vi "generate and convert rnd 1,2,3-D arrays.vi"(0 "dims":i32, 1 "numeric type const":T1, 5 "Tag":string, 9 "sizes":T4, 11 "error in (no error)":errorcluster) -> (2 "current timepoint":dbl, 3 "Array 1D":cdb[](array[numeric]), 4 "Array 2D":cdb[][](array[numeric]), 6 "Array 3D":cdb[][][](array[numeric]), 8 "bytes":i32, 10 "array as variant":variant, 12 "element size (bytes)":u8, 13 "delta t (s)":dbl, 14 "Bindata & descr out":T2, 15 "error out":errorcluster)   [LabVIEW 2018, in "LV2Julia_examples.lvlib"] (continued)
  1ec9265c-e1ac-4cb5-8500-03f8ca54a804.vi/ab8334bc-80fe-49a7-aeaa-72d4d4d986e9.vi/b9ff3e0a-05c7-4d11-a75b-368fec092445.vi/274aa64d-7dbc-4001-99d2-75c7e6616095.vi
  1ec9265c-e1ac-4cb5-8500-03f8ca54a804.vi/96353e94-dd23-4035-8dd4-90333fc8a4d3.vi/f4ce16f9-675e-447e-8c5f-32c7ef14206e.vi/2ab18f9f-d25e-4d6f-a422-5d1976ace012.vi
  1ec9265c-e1ac-4cb5-8500-03f8ca54a804.vi/167585a2-6b26-4dd4-a205-ebd7312b44a1.vi/4f7bf506-ab24-41ce-b71a-8160a5476407.vi/342633a8-57f8-4cc5-bcb8-03c25e82ca19.vi
  9cd03b83-d5bc-4a7f-9dd3-ef622f64ee30.vi/c26303ed-4f99-4591-9769-7eebad8d47fd.vi/1b763a9f-5ce5-41ba-bc7f-9f995f4d2b4d.vi/1789e023-f5c5-4665-87e0-2a6614aebc85.vi
  9cd03b83-d5bc-4a7f-9dd3-ef622f64ee30.vi/401e3ff0-0d76-40e6-a2f4-d101c51ec70e.vi/66e2e3b0-dc28-4f05-a834-250e6508c857.vi/552213f3-3728-4a7f-86dc-322237ece7cd.vi
  9cd03b83-d5bc-4a7f-9dd3-ef622f64ee30.vi/b4056afe-3c0d-4dbc-a3cd-b11ce2b05076.vi/40f3e5bb-f60e-451c-8b00-4309ab568451.vi/4e93cb2a-2fda-4bca-9a11-733b7b362d86.vi
  ee83ef70-773d-469c-ba23-25239dc81b12.vi/c87a68b0-2172-4a67-a6f0-f210c7451bd3.vi/84a80026-1c80-486c-8d92-8831a7df5ff3.vi/628bd820-375e-420b-b97f-d572ea6ad967.vi
  ee83ef70-773d-469c-ba23-25239dc81b12.vi/4135ce50-1702-49d5-b7b5-9d498c87c660.vi/d1bc0e7f-a379-4ff9-bf17-9e41a0f46a57.vi/980bb05f-dadf-4b86-b249-59f560e02473.vi
  ee83ef70-773d-469c-ba23-25239dc81b12.vi/9914fa42-08c7-43b8-a27e-b62889b56e78.vi/5de439e2-5012-4648-894c-bb1b9ad5bb26.vi/d9b0be4b-4247-47fe-91b4-82206086a95d.vi
  fca8e823-b190-45b9-9fbf-0f97a3b8de28.vi/a46cdcc9-52d0-4030-83dd-4ce08d19186e.vi/90bccda5-6ac7-4d46-9afb-e6399bdb2e1f.vi/078c7d38-6c67-4563-ab55-40eabe55752b.vi
  fca8e823-b190-45b9-9fbf-0f97a3b8de28.vi/4dbc5799-ec76-42b3-bb12-e906c396b96b.vi/ec007a79-76e9-41e5-8892-0302a9e6b40b.vi/301a90ca-8247-4ad5-ba2b-678751a04883.vi
  fca8e823-b190-45b9-9fbf-0f97a3b8de28.vi/cb420030-84f1-4efb-80b2-f5620303c743.vi/2c209796-9244-4d59-a9f5-eb5b4e6512ff.vi/25dea5f7-681f-4e0e-85cf-2491529aaee2.vi
  e5719774-7c0b-4606-b38f-adf2a3fe0ebf.vi/e04a025a-b044-48ec-9ce3-537d6650ec9f.vi/be8c913f-5955-4425-929d-934409af2b49.vi/d34738e1-42d1-4bf7-9a84-ddff0b876cf5.vi
  e5719774-7c0b-4606-b38f-adf2a3fe0ebf.vi/6399dd36-c1e6-41ee-ae47-d998c15f331f.vi/49d2f734-92bf-43e0-a325-d114aa2d52b5.vi/f6894c85-aa94-43f5-b724-8f72549e5cda.vi
  e5719774-7c0b-4606-b38f-adf2a3fe0ebf.vi/c5e050e8-c7cb-4905-8055-5f2d77b4ebae.vi/22426407-5a39-4ae1-b419-51b886c4e6cc.vi/0f5aa2a8-f382-4938-b1c0-af64f89efd9d.vi
  0f763169-7436-48fd-a14e-d5e7c7a3701c.vi/4318b9fa-7e96-4320-ad14-e58bf08cbdca.vi/ec80edef-ad4d-481c-bae0-ad236ad91d17.vi/99c98c4d-5a9d-4194-a764-b16bcb65aadc.vi
  0f763169-7436-48fd-a14e-d5e7c7a3701c.vi/42337aaa-b56a-45f8-8fc1-26a400602ff7.vi/853c4e43-66a7-4fd6-8a67-725115d20b02.vi/e1340f66-9321-4958-baeb-f40ca0670b2a.vi
  0f763169-7436-48fd-a14e-d5e7c7a3701c.vi/6ec92a7e-3200-4835-a3af-72f6deb2a7de.vi/d7fa0239-54ab-48c8-b35d-0719727c3c46.vi/a08a90ec-3f4e-4bf9-bfc8-c8b0dc2424f1.vi
  85ae8d2b-1833-426f-a7e3-0aa59edb462e.vi/8e85eddd-eeb1-48c7-aa0c-acb2476f15c2.vi/08ea7271-58f7-4381-bb13-89612bf68987.vi/c319c975-6598-4c49-9112-e1ac8bec7b87.vi/58ceea13-0e9b-4af9-9c64-6ddff0cfcc70.vi
  85ae8d2b-1833-426f-a7e3-0aa59edb462e.vi/af9a9771-594c-4ddf-b656-7825023e47e7.vi/a558cd4b-dbd0-4514-827e-24ca6e6b3a91.vi/23666670-5fa0-4551-929a-5078f8c88eb4.vi/ef739d47-3b07-40f6-99d3-e1375b6b8ec0.vi
  85ae8d2b-1833-426f-a7e3-0aa59edb462e.vi/f9469cc9-c20f-42ad-af32-5d4df993a375.vi/8c409728-000f-45f8-9ccd-ee15c7ed8521.vi/af52c658-7aca-4654-a19b-bdc00d5bce4f.vi/47bd8f68-fb6a-411a-b5e7-9fbf321a4e11.vi
  b7a12c6c-f00d-43e6-9642-9243e32b2058.vi/0ada88ee-c4f2-4d17-bb7a-74a21d7765a4.vi/69bbc40a-c36a-4917-aaee-edada7b7b8d7.vi/c11b2df1-177a-40a7-9ba6-98232f8d7f99.vi/7a8a583f-169c-44ac-bc13-e659061e41ae.vi
  b7a12c6c-f00d-43e6-9642-9243e32b2058.vi/502a5a5e-5782-46f9-888a-3583fb3fbf86.vi/571e470d-9707-4b89-9631-5b8d9304f753.vi/e1749920-efd2-42e0-885b-7fb6c4c5ab43.vi/a2170132-eaf3-4ab4-8383-804d572dbb60.vi
  b7a12c6c-f00d-43e6-9642-9243e32b2058.vi/963765af-ec1a-4af6-8576-dda3e1cb1b45.vi/a9e7bee4-94d8-4d8e-b190-a2971037c66e.vi/1f67fc8e-8653-4e8b-a6c2-2cf9980ddd08.vi/c5ad99fd-dcdc-41c3-9a54-18b338f6f827.vi
  ba780daf-ef06-44ce-bff3-6c34795b2ca8.vi/faf0b0c0-115a-4e37-90b8-e50dcc4168bc.vi/ff37c594-a005-47f5-bb34-4c70a0126acb.vi/c6e85278-50f0-4f6a-9193-dc1bcd0ef70f.vi/a77b55b7-d308-4fb3-aa63-6804bc56a6d7.vi
  ba780daf-ef06-44ce-bff3-6c34795b2ca8.vi/3ee41887-da2e-4051-ad5a-82b4c75e16db.vi/43312af0-9a58-49ee-9340-b8aa225bd272.vi/3269ca27-2cba-45df-9346-92c5d96bd6fc.vi/8956672e-b90e-41c9-981a-392c13e15a59.vi
  ba780daf-ef06-44ce-bff3-6c34795b2ca8.vi/440f1969-f94a-49e7-92dd-969720926e87.vi/1b453ea8-962a-4255-a994-0cbca27764d4.vi/f62144a5-f5db-4e00-a07d-a8ab4245d2e0.vi/63c49d2f-fa43-4a67-9b23-eadd08c82c33.vi
  0827bc69-4216-4d70-a1a4-4bfc71e08fdd.vi/261e91eb-d6ba-4368-8adb-b056b6d5af16.vi/d1f6d98c-0505-4e61-9b8c-a3eed1ff26ed.vi/7d30ac35-157d-4fcc-9b6f-176c22041dd3.vi/6365f774-6091-4c03-be79-b53c3a463edd.vi
  0827bc69-4216-4d70-a1a4-4bfc71e08fdd.vi/1cb40332-89ee-4e85-bdd1-f055d6e9593b.vi/3667db32-83c2-4485-8485-501a99b88cfe.vi/a5ed325d-485e-44f9-b4a5-b94842094a7d.vi/bbb4fa19-a19e-4b4f-a972-0fad6acc7987.vi
  0827bc69-4216-4d70-a1a4-4bfc71e08fdd.vi/2aac3158-face-4bd6-b9ad-b375428daa75.vi/10b5fca0-4c2a-4c9a-8b53-fb3dcff5ab00.vi/83375121-0e11-44d4-aa51-0de5076e5d92.vi/8d656ec8-2c6e-4c54-b472-f9621b7bc254.vi
  31a52eb7-4f60-473e-a06e-05ec52e66b84.vi/833f7a80-f94e-40d2-8863-3d22036f4c05.vi/de0d82be-3b4d-4b69-b774-1ee66ef3b500.vi/3a45cae5-de8a-427f-805d-7805f64916c3.vi/779167f3-7191-404e-9479-d306974a1702.vi
  31a52eb7-4f60-473e-a06e-05ec52e66b84.vi/4dc64207-d105-4bdf-b337-3f5f3ae1db54.vi/7b76e6e9-99fc-48fe-88e5-663e33f1532b.vi/06f57519-d6ad-4a96-9600-46d432553020.vi/86d7e16d-a525-46dc-8e9b-8a765bb4fd8a.vi
  31a52eb7-4f60-473e-a06e-05ec52e66b84.vi/caebaab9-5afa-4ebd-88ee-492fb4ee9da6.vi/ae77f17b-7a63-49d8-8677-2eb378eecda7.vi/07361902-21c8-49bd-b0fa-bce76e827913.vi/6519da9f-9d74-43b4-95c4-6905f871aa2b.vi
  be087227-1c24-4c50-b280-a6b288463f93.vi/77d648b1-c2bd-47e8-9d98-d5979e8947bd.vi/eb2ac645-ddc7-47bc-9d8b-75952129f04e.vi/90e6bd1a-94b1-4e35-a711-208e6fb95ce0.vi/4cf44929-3de7-4a16-8e6d-ba3e81e4c27d.vi
  be087227-1c24-4c50-b280-a6b288463f93.vi/9db986cd-cad9-4629-9f04-d611e563b09c.vi/b1da1a18-7165-4dcd-a4ff-b5fd07c18a7e.vi/e9ab5a05-9916-45bc-bc4c-428d98bb0cc0.vi/87e8c9e4-61f1-41fd-91f0-278c7c3c04e0.vi
  be087227-1c24-4c50-b280-a6b288463f93.vi/67544f08-8803-4e76-831f-e149eee3dcfb.vi/541c202c-62e7-4b26-a949-153a4b69c346.vi/04e1edd0-f714-4231-8a6f-30cd0f5f9b80.vi/a19ed12b-7c03-4017-abb4-26d2a47e06df.vi
  1496614b-dcbf-47d4-84ca-bd6c1ad99fe0.vi/47715fe6-eadc-4bbe-9722-e67c6229c693.vi/0fdc2738-6627-4de2-9d66-c6113426bbea.vi/30918f85-42e6-4e48-8a75-a92bfcdedf97.vi/d18d07c2-63c4-4e17-8723-4ec8b6dbf592.vi
  1496614b-dcbf-47d4-84ca-bd6c1ad99fe0.vi/8a8a2384-441c-4f35-bc10-b3d32a1405b6.vi/9880d032-961f-4e8d-bd85-807a3cb9978c.vi/30cf2ff2-8458-4241-b44f-73b870a3098c.vi/d1494cf9-d2bc-481b-b450-d9b2c9e1edeb.vi
  1496614b-dcbf-47d4-84ca-bd6c1ad99fe0.vi/a5d379dd-b135-4ded-bacd-aaa1ef77f126.vi/d1569549-6e2f-4408-83e1-6f356c70d908.vi/aa36f776-024c-45ea-9348-02a91e581604.vi/1736647a-b315-4943-a23a-7b6bb0983d47.vi
  1ec9265c-e1ac-4cb5-8500-03f8ca54a804.vi/ab8334bc-80fe-49a7-aeaa-72d4d4d986e9.vi/b9ff3e0a-05c7-4d11-a75b-368fec092445.vi/274aa64d-7dbc-4001-99d2-75c7e6616095.vi/3031d146-c71f-4ccc-b559-d2eec49110a8.vi
  1ec9265c-e1ac-4cb5-8500-03f8ca54a804.vi/96353e94-dd23-4035-8dd4-90333fc8a4d3.vi/f4ce16f9-675e-447e-8c5f-32c7ef14206e.vi/2ab18f9f-d25e-4d6f-a422-5d1976ace012.vi/7fef43ff-eeec-440e-9227-3c546e2cf6b2.vi
  1ec9265c-e1ac-4cb5-8500-03f8ca54a804.vi/167585a2-6b26-4dd4-a205-ebd7312b44a1.vi/4f7bf506-ab24-41ce-b71a-8160a5476407.vi/342633a8-57f8-4cc5-bcb8-03c25e82ca19.vi/f9b3a876-a45b-4cfa-ba65-04fa4f403bbb.vi
  9cd03b83-d5bc-4a7f-9dd3-ef622f64ee30.vi/c26303ed-4f99-4591-9769-7eebad8d47fd.vi/1b763a9f-5ce5-41ba-bc7f-9f995f4d2b4d.vi/1789e023-f5c5-4665-87e0-2a6614aebc85.vi/bb2d76ea-fe51-44ee-98c8-3538eddbe8f7.vi
  9cd03b83-d5bc-4a7f-9dd3-ef622f64ee30.vi/401e3ff0-0d76-40e6-a2f4-d101c51ec70e.vi/66e2e3b0-dc28-4f05-a834-250e6508c857.vi/552213f3-3728-4a7f-86dc-322237ece7cd.vi/2ae5eaef-0630-4360-94ee-a90142495add.vi
  9cd03b83-d5bc-4a7f-9dd3-ef622f64ee30.vi/b4056afe-3c0d-4dbc-a3cd-b11ce2b05076.vi/40f3e5bb-f60e-451c-8b00-4309ab568451.vi/4e93cb2a-2fda-4bca-9a11-733b7b362d86.vi/9563dd2e-97a5-4964-a1e0-f91578157d44.vi
  ee83ef70-773d-469c-ba23-25239dc81b12.vi/c87a68b0-2172-4a67-a6f0-f210c7451bd3.vi/84a80026-1c80-486c-8d92-8831a7df5ff3.vi/628bd820-375e-420b-b97f-d572ea6ad967.vi/1c6b066d-5cc1-4c38-ab51-bda082b626b1.vi
  ee83ef70-773d-469c-ba23-25239dc81b12.vi/4135ce50-1702-49d5-b7b5-9d498c87c660.vi/d1bc0e7f-a379-4ff9-bf17-9e41a0f46a57.vi/980bb05f-dadf-4b86-b249-59f560e02473.vi/b4362857-e7ba-464c-ae1c-547460d16cc5.vi
  ee83ef70-773d-469c-ba23-25239dc81b12.vi/9914fa42-08c7-43b8-a27e-b62889b56e78.vi/5de439e2-5012-4648-894c-bb1b9ad5bb26.vi/d9b0be4b-4247-47fe-91b4-82206086a95d.vi/7a7d3ea9-b799-4941-84ac-db74242acac8.vi
  fca8e823-b190-45b9-9fbf-0f97a3b8de28.vi/a46cdcc9-52d0-4030-83dd-4ce08d19186e.vi/90bccda5-6ac7-4d46-9afb-e6399bdb2e1f.vi/078c7d38-6c67-4563-ab55-40eabe55752b.vi/207eb310-9d0f-4098-b29f-a81cd0f1ec7c.vi
  fca8e823-b190-45b9-9fbf-0f97a3b8de28.vi/4dbc5799-ec76-42b3-bb12-e906c396b96b.vi/ec007a79-76e9-41e5-8892-0302a9e6b40b.vi/301a90ca-8247-4ad5-ba2b-678751a04883.vi/760c868c-a60a-4c7f-898c-61962456574a.vi
  fca8e823-b190-45b9-9fbf-0f97a3b8de28.vi/cb420030-84f1-4efb-80b2-f5620303c743.vi/2c209796-9244-4d59-a9f5-eb5b4e6512ff.vi/25dea5f7-681f-4e0e-85cf-2491529aaee2.vi/d8b50a02-5a58-479d-a4d1-5d953e0152d5.vi
  e5719774-7c0b-4606-b38f-adf2a3fe0ebf.vi/e04a025a-b044-48ec-9ce3-537d6650ec9f.vi/be8c913f-5955-4425-929d-934409af2b49.vi/d34738e1-42d1-4bf7-9a84-ddff0b876cf5.vi/cdb26c22-a524-4e5d-b25f-6c6bd3956a64.vi
  e5719774-7c0b-4606-b38f-adf2a3fe0ebf.vi/6399dd36-c1e6-41ee-ae47-d998c15f331f.vi/49d2f734-92bf-43e0-a325-d114aa2d52b5.vi/f6894c85-aa94-43f5-b724-8f72549e5cda.vi/c88dc2f1-b7ef-422b-a2cc-e5b0aafc2ba8.vi
  e5719774-7c0b-4606-b38f-adf2a3fe0ebf.vi/c5e050e8-c7cb-4905-8055-5f2d77b4ebae.vi/22426407-5a39-4ae1-b419-51b886c4e6cc.vi/0f5aa2a8-f382-4938-b1c0-af64f89efd9d.vi/61b47ad3-8083-4dfa-9844-e0f84142c628.vi
  0f763169-7436-48fd-a14e-d5e7c7a3701c.vi/4318b9fa-7e96-4320-ad14-e58bf08cbdca.vi/ec80edef-ad4d-481c-bae0-ad236ad91d17.vi/99c98c4d-5a9d-4194-a764-b16bcb65aadc.vi/5a9aa0de-9cb3-4491-9cf7-b27116c16558.vi
  0f763169-7436-48fd-a14e-d5e7c7a3701c.vi/42337aaa-b56a-45f8-8fc1-26a400602ff7.vi/853c4e43-66a7-4fd6-8a67-725115d20b02.vi/e1340f66-9321-4958-baeb-f40ca0670b2a.vi/fe3983ef-dbb8-4cc1-bf41-859b9b1c4fd8.vi
  0f763169-7436-48fd-a14e-d5e7c7a3701c.vi/6ec92a7e-3200-4835-a3af-72f6deb2a7de.vi/d7fa0239-54ab-48c8-b35d-0719727c3c46.vi/a08a90ec-3f4e-4bf9-bfc8-c8b0dc2424f1.vi/d5c99d08-ae4e-4c5e-a5fb-c6e0d147efb0.vi
  LV2Julia_core/VIs/check ID validity.vi
  LV2Julia_core/VIs/rnd(span).vi
  LV2Julia_core/LV2Julia_core.lvlib
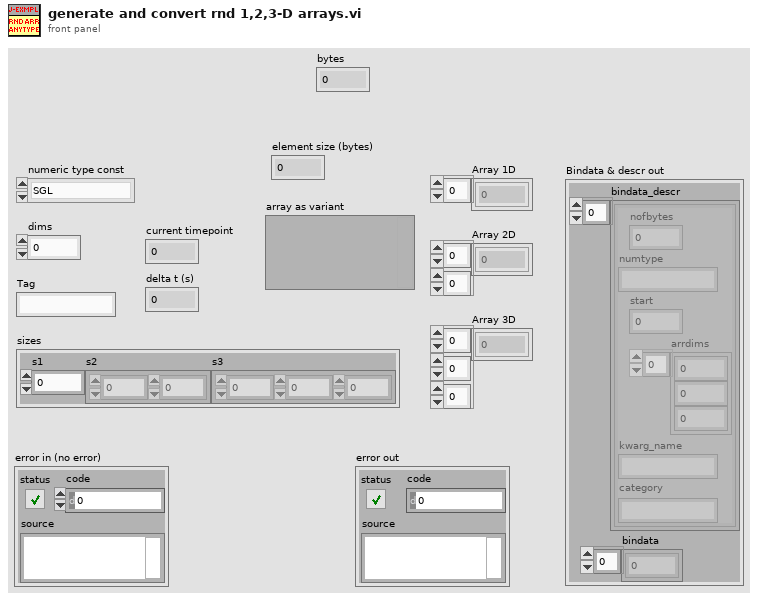
[diagram p1: front panel]
types:
  T1 = typedef "LV2Julia_core.lvlib/Numeric Types enum.ctl" = enum16{"SGL", "DBL", "I8", "I16", "I32", "I64", "U8", "U16", "U32", "U64", "CSGL", "CDBL", "boolean"}
  T2 = typedef "LV2Julia_core.lvlib/Bindata&description.ctl" = cluster{"bindata_descr":T3[], "bindata":u8[]}
  T3 = typedef "LV2Julia_core.lvlib/Bindata description.ctl" = cluster{"nofbytes":i32, "numtype":string, "start":i32, "arrdims":i32[], "kwarg_name":string, "category":string}
  T4 = typedef "LV2Julia_examples.lvlib/array 123D sizes.ctl" = cluster{"s1":i32, "s2":i32[], "s3":i32[]}
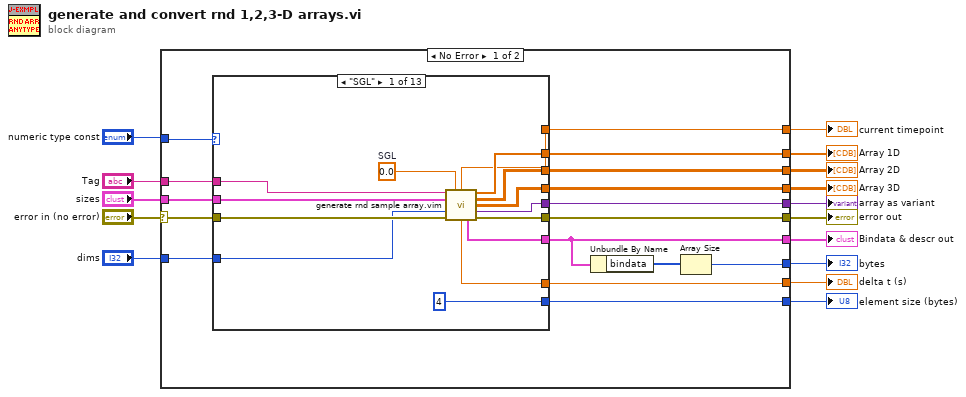
[diagram p0: block diagram]
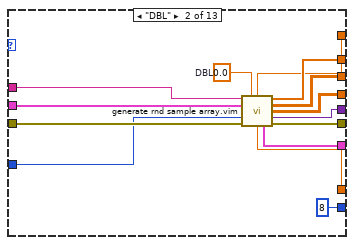
[diagram p2: hidden frame]
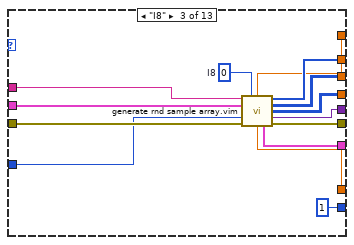
[diagram p3: hidden frame]
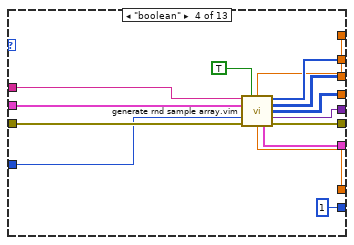
[diagram p4: hidden frame]
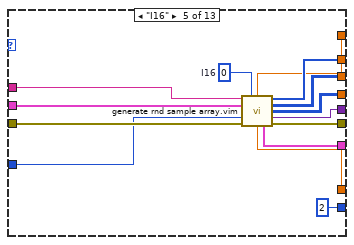
[diagram p5: hidden frame]
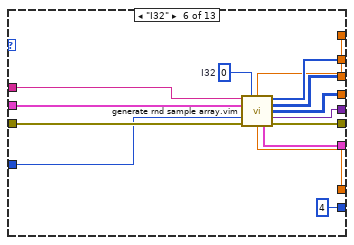
[diagram p6: hidden frame]
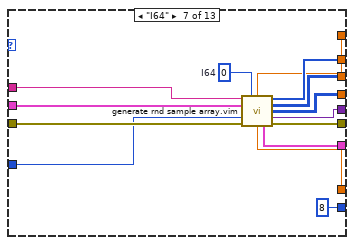
[diagram p7: hidden frame]
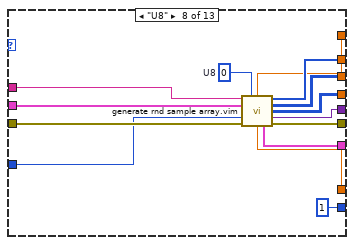
[diagram p8: hidden frame]
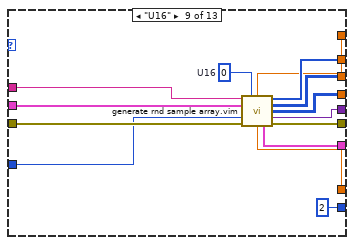
[diagram p9: hidden frame]
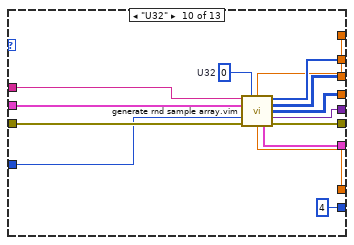
[diagram p10: hidden frame]
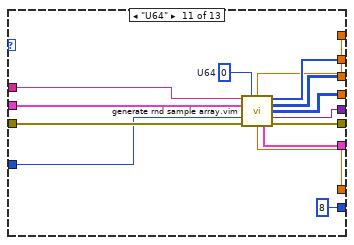
[diagram p11: hidden frame]
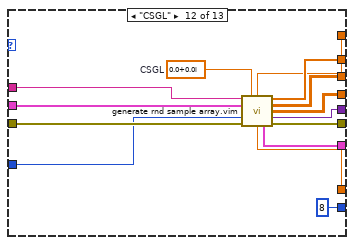
[diagram p12: hidden frame]
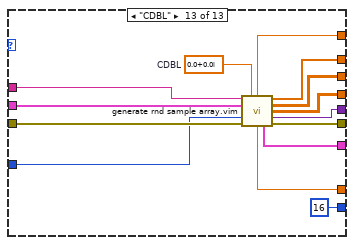
[diagram p13: hidden frame]
diagram:
  n1 = case shown="No Error" "error in (no error)" {
    selector: "error in (no error)" -> [w26 w214]
    tunnel: [w31 w214] -> w15
    tunnel: [w18 _] -> w12
    tunnel: "Tag" -> [w30 _]
    tunnel: [w29 _] -> w4
    tunnel: "numeric type const" -> [w28 _]
    tunnel: "dims" -> [w27 _]
    tunnel: [w25 _] -> w9
    tunnel: [w24 _] -> w10
    tunnel: [w23 _] -> w11
    tunnel: "sizes" -> [w22 _]
    tunnel: [w21 _] -> w14
    tunnel: [w20 _] -> w3
    tunnel: [w19 _] -> w2
    tunnel: [w16 _] -> w1
    frame No Error {
      n2 = case shown="\"SGL\"" w28 {
        tunnel: [w45 w59 w73 w87 w101 w115 w129 w143 w157 w171 w185 w199 w213] -> w31
        tunnel: [w44 w58 w72 w86 w100 w114 w128 w142 w156 w170 w184 w198 w212] -> w18
        tunnel: w26 -> [w43 w57 w71 w85 w99 w113 w127 w141 w155 w169 w183 w197 w211]
        tunnel: w27 -> [w42 w56 w70 w84 w98 w112 w126 w140 w154 w168 w182 w196 w210]
        tunnel: w30 -> [w41 w55 w69 w83 w97 w111 w125 w139 w153 w167 w181 w195 w209]
        tunnel: [w39 w53 w67 w82 w95 w109 w123 w137 w151 w165 w179 w193 w207] -> w29
        tunnel: [w38 w50 w64 w79 w92 w106 w120 w134 w148 w162 w176 w190 w204] -> w23
        tunnel: [w37 w51 w65 w80 w93 w107 w121 w135 w149 w163 w177 w191 w205] -> w24
        tunnel: [w36 w52 w66 w81 w94 w108 w122 w136 w150 w164 w178 w192 w206] -> w25
        tunnel: w22 -> [w35 w49 w63 w77 w91 w105 w119 w133 w147 w161 w175 w189 w203]
        tunnel: [w34 w48 w62 w76 w90 w104 w118 w132 w146 w160 w174 w188 w202] -> w21
        tunnel: [w33 w47 w61 w75 w89 w103 w117 w131 w145 w159 w173 w187 w201] -> w20
        tunnel: [u8 4 u8 8 u8 1 u8 1 u8 2 u8 4 u8 8 u8 1 u8 2 u8 4 u8 8 u8 8 u8 16] -> w19
        frame "SGL" {
          w40 = sgl 0.0  # SGL
          n3 = call "generate rnd sample array.vim"("kwarg_name"=w41, "type"=w40, "array sizes"=w35, "dims"=w42, "error in (no error)"=w43) -> ("current timepoint"=w33:dbl, "Array 1D"=w36:sgl[], "Array 2D"=w37:sgl[][], "Array 3D"=w38:sgl[][][], "array as variant"=w39:variant, "delta t (s)"=w34:dbl, "Bindata & descr out"=w44:T2, "error out"=w45:errorcluster)  [unwired: 2 in, 1 out]
        }
        frame "DBL" {
          w54 = 0.0  # DBL
          n4 = call "generate rnd sample array.vim"("kwarg_name"=w55, "type"=w54, "array sizes"=w49, "dims"=w56, "error in (no error)"=w57) -> ("current timepoint"=w47:dbl, "Array 1D"=w52:dbl[], "Array 2D"=w51:dbl[][], "Array 3D"=w50:dbl[][][], "array as variant"=w53:variant, "delta t (s)"=w48:dbl, "Bindata & descr out"=w58:T2, "error out"=w59:errorcluster)  [unwired: 2 in, 1 out]
        }
        frame "I8" {
          w68 = i8 0  # I8
          n5 = call "generate rnd sample array.vim"("kwarg_name"=w69, "type"=w68, "array sizes"=w63, "dims"=w70, "error in (no error)"=w71) -> ("current timepoint"=w61:dbl, "Array 1D"=w66:i8[], "Array 2D"=w65:i8[][], "Array 3D"=w64:i8[][][], "array as variant"=w67:variant, "delta t (s)"=w62:dbl, "Bindata & descr out"=w72:T2, "error out"=w73:errorcluster)  [unwired: 2 in, 1 out]
        }
        frame "boolean" {
          n6 = call "generate rnd sample array.vim"("kwarg_name"=w83, "type"=TRUE, "array sizes"=w77, "dims"=w84, "error in (no error)"=w85) -> ("current timepoint"=w75:dbl, "Array 1D"=w81:i16[], "Array 2D"=w80:i16[][], "Array 3D"=w79:i16[][][], "array as variant"=w82:variant, "delta t (s)"=w76:dbl, "Bindata & descr out"=w86:T2, "error out"=w87:errorcluster)  [unwired: 2 in, 1 out]
        }
        frame "I16" {
          w96 = i16 0  # I16
          n7 = call "generate rnd sample array.vim"("kwarg_name"=w97, "type"=w96, "array sizes"=w91, "dims"=w98, "error in (no error)"=w99) -> ("current timepoint"=w89:dbl, "Array 1D"=w94:i16[], "Array 2D"=w93:i16[][], "Array 3D"=w92:i16[][][], "array as variant"=w95:variant, "delta t (s)"=w90:dbl, "Bindata & descr out"=w100:T2, "error out"=w101:errorcluster)  [unwired: 2 in, 1 out]
        }
        frame "I32" {
          w110 = 0  # I32
          n8 = call "generate rnd sample array.vim"("kwarg_name"=w111, "type"=w110, "array sizes"=w105, "dims"=w112, "error in (no error)"=w113) -> ("current timepoint"=w103:dbl, "Array 1D"=w108:i32[], "Array 2D"=w107:i32[][], "Array 3D"=w106:i32[][][], "array as variant"=w109:variant, "delta t (s)"=w104:dbl, "Bindata & descr out"=w114:T2, "error out"=w115:errorcluster)  [unwired: 2 in, 1 out]
        }
        frame "I64" {
          w124 = i64 0  # I64
          n9 = call "generate rnd sample array.vim"("kwarg_name"=w125, "type"=w124, "array sizes"=w119, "dims"=w126, "error in (no error)"=w127) -> ("current timepoint"=w117:dbl, "Array 1D"=w122:i64[], "Array 2D"=w121:i64[][], "Array 3D"=w120:i64[][][], "array as variant"=w123:variant, "delta t (s)"=w118:dbl, "Bindata & descr out"=w128:T2, "error out"=w129:errorcluster)  [unwired: 2 in, 1 out]
        }
        frame "U8" {
          w138 = u8 0  # U8
          n10 = call "generate rnd sample array.vim"("kwarg_name"=w139, "type"=w138, "array sizes"=w133, "dims"=w140, "error in (no error)"=w141) -> ("current timepoint"=w131:dbl, "Array 1D"=w136:u8[], "Array 2D"=w135:u8[][], "Array 3D"=w134:u8[][][], "array as variant"=w137:variant, "delta t (s)"=w132:dbl, "Bindata & descr out"=w142:T2, "error out"=w143:errorcluster)  [unwired: 2 in, 1 out]
        }
        frame "U16" {
          w152 = u16 0  # U16
          n11 = call "generate rnd sample array.vim"("kwarg_name"=w153, "type"=w152, "array sizes"=w147, "dims"=w154, "error in (no error)"=w155) -> ("current timepoint"=w145:dbl, "Array 1D"=w150:u16[], "Array 2D"=w149:u16[][], "Array 3D"=w148:u16[][][], "array as variant"=w151:variant, "delta t (s)"=w146:dbl, "Bindata & descr out"=w156:T2, "error out"=w157:errorcluster)  [unwired: 2 in, 1 out]
        }
        frame "U32" {
          w166 = u32 0  # U32
          n12 = call "generate rnd sample array.vim"("kwarg_name"=w167, "type"=w166, "array sizes"=w161, "dims"=w168, "error in (no error)"=w169) -> ("current timepoint"=w159:dbl, "Array 1D"=w164:u32[], "Array 2D"=w163:u32[][], "Array 3D"=w162:u32[][][], "array as variant"=w165:variant, "delta t (s)"=w160:dbl, "Bindata & descr out"=w170:T2, "error out"=w171:errorcluster)  [unwired: 2 in, 1 out]
        }
        frame "U64" {
          w180 = u64 0  # U64
          n13 = call "generate rnd sample array.vim"("kwarg_name"=w181, "type"=w180, "array sizes"=w175, "dims"=w182, "error in (no error)"=w183) -> ("current timepoint"=w173:dbl, "Array 1D"=w178:u64[], "Array 2D"=w177:u64[][], "Array 3D"=w176:u64[][][], "array as variant"=w179:variant, "delta t (s)"=w174:dbl, "Bindata & descr out"=w184:T2, "error out"=w185:errorcluster)  [unwired: 2 in, 1 out]
        }
        frame "CSGL" {
          w194 = csg 0.0+0.0i  # CSGL
          n14 = call "generate rnd sample array.vim"("kwarg_name"=w195, "type"=w194, "array sizes"=w189, "dims"=w196, "error in (no error)"=w197) -> ("current timepoint"=w187:dbl, "Array 1D"=w192:csg[], "Array 2D"=w191:csg[][], "Array 3D"=w190:csg[][][], "array as variant"=w193:variant, "delta t (s)"=w188:dbl, "Bindata & descr out"=w198:T2, "error out"=w199:errorcluster)  [unwired: 2 in, 1 out]
        }
        frame "CDBL" {
          w208 = cdb 0.0+0.0i  # CDBL
          n15 = call "generate rnd sample array.vim"("kwarg_name"=w209, "type"=w208, "array sizes"=w203, "dims"=w210, "error in (no error)"=w211) -> ("current timepoint"=w201:dbl, "Array 1D"=w206:cdb[], "Array 2D"=w205:cdb[][], "Array 3D"=w204:cdb[][][], "array as variant"=w207:variant, "delta t (s)"=w202:dbl, "Bindata & descr out"=w212:T2, "error out"=w213:errorcluster)  [unwired: 2 in, 1 out]
        }
      }
      n16 = Unbundle By Name(w18) -> ("bindata"=w17:u8[])
      n17 = Array Size(array=w17) -> (size(s)=w16:i32)
    }
    frame Error {
    }
  }
  "error out" <- w15
  "delta t (s)" <- w14
  "Bindata & descr out" <- w12
  "Array 3D" <- w11
  "Array 2D" <- w10
  "Array 1D" <- w9
  "array as variant" <- w4
  "current timepoint" <- w3
  "element size (bytes)" <- w2
  "bytes" <- w1
